vi "Dresden R2R Sputter 03.02.2018 IY24.vi"() -> ()   [LabVIEW 2009] (continued)
                                }
                                }
                                n29425 = Or(x=w34352, y=w34351) -> (x .or. y?=w34350:bool)
                                }
                                }
                                frame #1 {
                                }
                                }
                                }
                                frame #1 {
                                }
                                }
                                }
                                frame #4 {
                                n29426 = local read "Semi"() -> (w34358:bool)
                                n29427 = case shown="False" w34358 {
                                frame #0 {
                                n29428 = Wait (ms)(milliseconds to wait=u32 1000) -> ()  [unwired: 1 out]
                                }
                                frame #1 {
                                }
                                }
                                }
                                }
                                }
                                frame #1 {
                                }
                                }
                                }
                                frame #1 {
                                n29429 = local read "Semi"() -> (w34360:bool)
                                n29430 = case shown="False" w34360 {
                                frame #0 {
                                n29431 = local write "SDC1 26"(TRUE ("SDC1 26")) -> ()
                                n29432 = Wait (ms)(milliseconds to wait=u32 1000) -> ()  [unwired: 1 out]
                                }
                                frame #1 {
                                }
                                }
                                }
                                }
                                }
                                frame #23 {
                                # "sov-ar close"
                                n29433 = stacked-sequence {
                                frame #0 {
                                n29434 = local read "Semi"() -> (w34363:bool)
                                n29435 = case shown="False" w34363 {
                                frame #0 {
                                n29436 = while {
                                i -> [w34369]
                                stop <- w34364 stop-if-true
                                n29437 = Greater?(x=w34369, y=50) -> (0:w34368:bool)
                                n29438 = case shown="True" w34368 {
                                frame #0 {
                                }
                                frame #1 {
                                n29439 = local write "Semi"(TRUE ("Semi")) -> ()
                                n29440 = local write "Error Message"("Coating Process  \nwas cancelled.\nPlease check \nSOV-Ar connection." ("Error Message")) -> ()
                                }
                                }
                                n29441 = local read "Ch4_Sov_Ar_di"() -> (w34367:bool)
                                n29442 = case shown="True" w34367 {
                                tunnel: [TRUE FALSE] -> w34366
                                frame #0 {
                                }
                                frame #1 {
                                n29443 = local write "Ch4_Sov_Ar_do"(FALSE ("Ch1_WFC_do")) -> ()
                                n29444 = Wait Until Next ms Multiple(millisecond multiple=u32 200) -> ()  [unwired: 1 out]
                                }
                                }
                                n29445 = local read "Semi"() -> (w34365:bool)
                                n29446 = Or(x=w34366, y=w34365) -> (x .or. y?=w34364:bool)
                                }
                                }
                                frame #1 {
                                }
                                }
                                }
                                frame #1 {
                                n29447 = local read "Semi"() -> (w34377:bool)
                                n29448 = case shown="False" w34377 {
                                frame #0 {
                                n29449 = local write "SDC1 27"(TRUE ("SDC1 27")) -> ()
                                n29450 = Wait (ms)(milliseconds to wait=u32 1000) -> ()  [unwired: 1 out]
                                }
                                frame #1 {
                                }
                                }
                                }
                                }
                                }
                                frame #24 {
                                # "CC OPEN"
                                n29451 = stacked-sequence {
                                frame #0 {
                                n29452 = local read "Semi"() -> (w34380:bool)
                                n29453 = case shown="False" w34380 {
                                frame #0 {
                                n29454 = while {
                                i -> [w34386]
                                stop <- w34381 stop-if-true
                                n29455 = Greater?(x=w34386, y=50) -> (0:w34385:bool)
                                n29456 = case shown="True" w34385 {
                                frame #0 {
                                }
                                frame #1 {
                                n29457 = local write "Semi"(TRUE ("Semi")) -> ()
                                n29458 = local write "Error Message"("Coating Process  \nwas cancelled.\nPlease check \nBG-BV connection." ("Error Message")) -> ()
                                }
                                }
                                n29459 = local read "Ch4_Cc_on_off_di"() -> (w34384:bool)
                                n29460 = case shown="False" w34384 {
                                tunnel: [FALSE TRUE] -> w34383
                                frame #0 {
                                n29461 = local write "Ch4_Cc_on_off_do"(TRUE ("Ch1_WFC_do")) -> ()
                                n29462 = Wait Until Next ms Multiple(millisecond multiple=u32 200) -> ()  [unwired: 1 out]
                                }
                                frame #1 {
                                }
                                }
                                n29463 = local read "Semi"() -> (w34382:bool)
                                n29464 = Or(x=w34383, y=w34382) -> (x .or. y?=w34381:bool)
                                }
                                }
                                frame #1 {
                                }
                                }
                                }
                                frame #1 {
                                n29465 = local read "Semi"() -> (w34394:bool)
                                n29466 = case shown="False" w34394 {
                                frame #0 {
                                n29467 = while {
                                i -> [w34399]
                                stop <- w34397 stop-if-true
                                n29468 = Greater?(x=w34399, y=30) -> (0:w34395:bool)
                                n29469 = Wait Until Next ms Multiple(millisecond multiple=u32 1000) -> ()  [unwired: 1 out]
                                n29470 = local read "Semi"() -> (w34398:bool)
                                n29471 = Or(x=w34395, y=w34398) -> (x .or. y?=w34397:bool)
                                }
                                }
                                frame #1 {
                                }
                                }
                                }
                                frame #2 {
                                n29472 = local read "Semi"() -> (w34401:bool)
                                n29473 = case shown="False" w34401 {
                                frame #0 {
                                n29474 = local write "SDC1 27b"(TRUE ("SDC1 3")) -> ()
                                n29475 = Wait (ms)(milliseconds to wait=u32 1000) -> ()  [unwired: 1 out]
                                }
                                frame #1 {
                                }
                                }
                                }
                                }
                                }
                                frame #25 {
                                # "CHECK CHAMBER PRESSURE"
                                n29476 = stacked-sequence {
                                frame #0 {
                                n29477 = local read "Semi"() -> (w34404:bool)
                                n29478 = case shown="False" w34404 {
                                frame #0 {
                                n29479 = while {
                                i -> [w34412]
                                stop <- w34406 stop-if-true
                                n29480 = Greater?(x=w34412, y=300) -> (0:w34411:bool)
                                n29481 = case shown="True" w34411 {
                                frame #0 {
                                }
                                frame #1 {
                                n29482 = local write "Semi"(TRUE ("Semi")) -> ()
                                n29483 = local write "Error Message"("Coating Process cancelled.\nPlease check chamber \nconnections." ("Error Message")) -> ()
                                }
                                }
                                n29484 = local read "Ch_CC_press_ch4_2"() -> (w34405:dbl)
                                n29485 = Greater Or Equal?(x=w34405, y=5e-05 ("CHAMBER PRESSURE 6")) -> (x >= y?=w34409:bool)
                                n29486 = case shown="True" w34409 {
                                tunnel: [TRUE FALSE] -> w34408
                                frame #0 {
                                }
                                frame #1 {
                                n29487 = Wait Until Next ms Multiple(millisecond multiple=u32 200) -> ()  [unwired: 1 out]
                                }
                                }
                                n29488 = local read "Semi"() -> (w34407:bool)
                                n29489 = Or(x=w34408, y=w34407) -> (x .or. y?=w34406:bool)
                                }
                                }
                                frame #1 {
                                }
                                }
                                }
                                frame #1 {
                                n29490 = local read "Semi"() -> (w34419:bool)
                                n29491 = case shown="False" w34419 {
                                frame #0 {
                                n29492 = Wait (ms)(milliseconds to wait=u32 1000) -> ()  [unwired: 1 out]
                                n29493 = local write "SDC1 27c"(TRUE ("SDC1 10")) -> ()
                                }
                                frame #1 {
                                }
                                }
                                }
                                }
                                }
                                frame #26 {
                                # "encoder info  add to other web selection"
                                n29494 = stacked-sequence {
                                frame #0 {
                                n29495 = local read "Semi"() -> (w34422:bool)
                                n29496 = case shown="False" w34422 {
                                frame #0 {
                                n29497 = local read "R_Web_selection"() -> (w34423:enum32{"Web", "Other"})
                                n29498 = case shown="\"Web\", Default" w34423 {
                                frame #0 {
                                # "TC -ROLL"
                                n29499 = local read "Semi"() -> (w34424:bool)
                                n29500 = case shown="False" w34424 {
                                frame #0 {
                                n29501 = stacked-sequence {
                                frame #0 {
                                n29502 = local read "R Maximum diameter"() -> (w34426:dbl)
                                n29503 = local write "Change_Max Diameter"(w34426) -> ()
                                n29504 = Wait (ms)(milliseconds to wait=u32 300) -> ()  [unwired: 1 out]
                                }
                                frame #1 {
                                n29505 = local read "R Single RF Step1 Coating Power Active"() -> (w34427:bool)
                                n29506 = local read "R Single RF Step2 Coating Power Active"() -> (w34428:bool)
                                n29507 = local read "R Single RF Step3 Coating Power Active"() -> (w34429:bool)
                                n29508 = local read "R Single RF Step4 Coating Power Active"() -> (w34430:bool)
                                n29509 = local read "R Single RF Step5 Coating Power Active"() -> (w34431:bool)
                                n29510 = Boolean To (0,1)(Boolean=w34427) -> (0, 1=w34432:i16)
                                n29511 = Boolean To (0,1)(Boolean=w34428) -> (0, 1=w34433:i16)
                                n29512 = Boolean To (0,1)(Boolean=w34429) -> (0, 1=w34434:i16)
                                n29513 = Boolean To (0,1)(Boolean=w34430) -> (0, 1=w34435:i16)
                                n29514 = Boolean To (0,1)(Boolean=w34431) -> (0, 1=w34436:i16)
                                n29515 = Compound Arithmetic op=ADD(w34432, w34433, w34434, w34435, w34436) -> (w34438:i16)
                                n29516 = local read "R Single RF Interval length"() -> (w34437:dbl)
                                n29517 = Multiply(x=w34437, y=w34438) -> (x*y=w34439:dbl)
                                n29518 = local write "Total length"(w34439) -> ()
                                }
                                frame #2 {
                                n29519 = local write "Calculate 3"(TRUE ("Calculate_auto")) -> ()
                                }
                                frame #3 {
                                n29520 = Wait (ms)(milliseconds to wait=u32 1000) -> ()  [unwired: 1 out]
                                }
                                frame #4 {
                                n29521 = local read "Change_Max Diameter"() -> (w34444:dbl)
                                n29522 = Wait (ms)(milliseconds to wait=u32 200) -> ()  [unwired: 1 out]
                                n29523 = local write "Web Speed"(200.0 ("Web Speed")) -> ()
                                n29524 = local write "Initial Min Diameter"(w34444) -> ()
                                }
                                frame #5 {
                                n29525 = local write "Calculate 2"(TRUE ("Calculate_auto")) -> ()
                                }
                                frame #6 {
                                n29526 = local write "Roll_side_select"(enum32{"Left to Right", "Right to Left"}."Right to Left" ("Roll_side_select")) -> ()
                                }
                                frame #7 {
                                n29527 = Wait (ms)(milliseconds to wait=u32 100) -> ()  [unwired: 1 out]
                                n29528 = local write "Parameters_auto_set"(TRUE ("Parameters_auto_set")) -> ()
                                }
                                frame #8 {
                                n29529 = while {
                                i -> [w34453]
                                stop <- w34449 stop-if-true
                                n29530 = Wait Until Next ms Multiple(millisecond multiple=u32 300) -> ()  [unwired: 1 out]
                                n29531 = Greater?(x=w34453, y=100) -> (0:w34450:bool)
                                n29532 = local read "Parameters_auto_set"() -> (w34454:bool)
                                n29533 = case shown="False" w34454 {
                                tunnel: [TRUE FALSE] -> w34451
                                frame #0 {
                                }
                                frame #1 {
                                }
                                }
                                n29534 = Or(x=w34451, y=w34450) -> (x .or. y?=w34449:bool)
                                }
                                }
                                frame #9 {
                                n29535 = local read "R Tension Value"() -> (w34458:dbl)
                                n29536 = Wait (ms)(milliseconds to wait=u32 200) -> ()  [unwired: 1 out]
                                n29537 = local write "TC2_set_value"(w34458) -> ()
                                }
                                frame #10 {
                                n29538 = local write "TC2_auto_set"(TRUE ("TC1_auto_set")) -> ()
                                }
                                frame #11 {
                                w34461 = u16 3 items=["1", "2", "3", "4"] ("Target Chamber Sensor")
                                n29539 = local write "Target Chamber Sensor"(w34461) -> ()
                                }
                                frame #12 {
                                n29540 = local read "Total length"() -> (w34462:dbl)
                                n29541 = local write "Region"(w34462) -> ()
                                }
                                frame #13 {
                                n29542 = local read "Semi"() -> (w34463:bool)
                                n29543 = case shown="False" w34463 {
                                frame #0 {
                                n29544 = local write "Start_roll"(TRUE ("Start_roll")) -> ()
                                n29545 = Wait (ms)(milliseconds to wait=u32 300) -> ()  [unwired: 1 out]
                                }
                                frame #1 {
                                }
                                }
                                }
                                frame #14 {
                                n29546 = local read "Semi"() -> (w34466:bool)
                                n29547 = case shown="False" w34466 {
                                frame #0 {
                                n29548 = while {
                                stop <- w34470 stop-if-true
                                n29549 = Wait Until Next ms Multiple(millisecond multiple=u32 200 ("milliseconds to wait")) -> ()  [unwired: 1 out]
                                n29550 = local read "Start_roll"() -> (w34468:bool)
                                n29551 = Not(x=w34468) -> (.not. x?=w34467:bool)
                                n29552 = local read "Semi"() -> (w34471:bool)
                                n29553 = Or(x=w34467, y=w34471) -> (x .or. y?=w34470:bool)
                                }
                                }
                                frame #1 {
                                }
                                }
                                }
                                }
                                }
                                frame #1 {
                                }
                                }
                                }
                                frame #1 {
                                n29554 = disable-structure shown="Disabled" {
                                frame #0 {
                                # "OTHER"
                                n29555 = local read "Semi"() -> (w34472:bool)
                                n29556 = case shown="False" w34472 {
                                frame #0 {
                                n29557 = stacked-sequence {
                                frame #0 {
                                n29558 = local read "Semi"() -> (w34473:bool)
                                n29559 = case shown="False" w34473 {
                                frame #0 {
                                n29560 = while {
                                i -> [w34479]
                                stop <- w34476 stop-if-true
                                n29561 = Greater?(x=w34479, y=50) -> (0:w34478:bool)
                                n29562 = case shown="True" w34478 {
                                frame #0 {
                                }
                                frame #1 {
                                n29563 = local write "Error Message"("" ("Error Message")) -> ()
                                n29564 = local write "Semi"(TRUE ("Semi")) -> ()
                                }
                                }
                                n29565 = local read "Casette_servo_start/stop_di"() -> (w34475:bool)
                                n29566 = case shown="False" w34475 {
                                tunnel: [FALSE TRUE] -> w34474
                                frame #0 {
                                n29567 = local write "Casette_servo_start/stop_do"(TRUE ("Casette_servo_left_direction_do")) -> ()
                                n29568 = Wait Until Next ms Multiple(millisecond multiple=u32 500) -> ()  [unwired: 1 out]
                                }
                                frame #1 {
                                }
                                }
                                n29569 = local read "Semi"() -> (w34477:bool)
                                n29570 = Or(x=w34474, y=w34477) -> (x .or. y?=w34476:bool)
                                }
                                }
                                frame #1 {
                                }
                                }
                                }
                                frame #1 {
                                n29571 = local read "Semi"() -> (w34487:bool)
                                n29572 = case shown="False" w34487 {
                                frame #0 {
                                n29573 = while {
                                i -> [w34493]
                                stop <- w34490 stop-if-true
                                n29574 = Greater?(x=w34493, y=50) -> (0:w34492:bool)
                                n29575 = case shown="True" w34492 {
                                frame #0 {
                                }
                                frame #1 {
                                n29576 = local write "Error Message"("" ("Error Message")) -> ()
                                n29577 = local write "Semi"(TRUE ("Semi")) -> ()
                                }
                                }
                                n29578 = local read "Casette_servo_left_direction_di"() -> (w34489:bool)
                                n29579 = case shown="False" w34489 {
                                tunnel: [FALSE TRUE] -> w34488
                                frame #0 {
                                n29580 = local write "Casette_servo_left_direction_do"(TRUE ("Casette_servo_left_direction_do")) -> ()
                                n29581 = Wait Until Next ms Multiple(millisecond multiple=u32 200) -> ()  [unwired: 1 out]
                                }
                                frame #1 {
                                }
                                }
                                n29582 = local read "Semi"() -> (w34491:bool)
                                n29583 = Or(x=w34488, y=w34491) -> (x .or. y?=w34490:bool)
                                }
                                }
                                frame #1 {
                                }
                                }
                                }
                                frame #2 {
                                # "casette motion"
                                n29584 = while {
                                i -> [w34503]
                                stop <- w34501 stop-if-true
                                n29585 = Greater?(x=w34503, y=200) -> (0:w34504:bool)
                                n29586 = case shown="True" w34504 {
                                frame #0 {
                                }
                                frame #1 {
                                n29587 = local write "Semi"(TRUE ("Semi")) -> ()
                                }
                                }
                                n29588 = local read "Counter_read_data"() -> (w34509:i16)
                                n29589 = Greater?(x=w34509, y=i16 0) -> (0:w34507:bool)
                                n29590 = case shown="True" w34507 {
                                tunnel: [TRUE TRUE] -> w34506
                                frame #0 {
                                }
                                frame #1 {
                                n29591 = local write "Casette_servo_start/stop_do"(FALSE ("Casette_servo_start/stop_do")) -> ()
                                n29592 = Wait Until Next ms Multiple(millisecond multiple=u32 200) -> ()  [unwired: 1 out]
                                }
                                }
                                n29593 = local read "Semi"() -> (w34505:bool)
                                n29594 = Or(x=w34506, y=w34505) -> (x .or. y?=w34501:bool)
                                }
                                }
                                frame #3 {
                                n29595 = local read "Semi"() -> (w34515:bool)
                                n29596 = case shown="False" w34515 {
                                frame #0 {
                                n29597 = while {
                                i -> [w34521]
                                stop <- w34518 stop-if-true
                                n29598 = Greater?(x=w34521, y=50) -> (0:w34520:bool)
                                n29599 = case shown="True" w34520 {
                                frame #0 {
                                }
                                frame #1 {
                                n29600 = local write "Error Message"("" ("Error Message")) -> ()
                                n29601 = local write "Semi"(TRUE ("Semi")) -> ()
                                }
                                }
                                n29602 = local read "Casette_servo_start/stop_di"() -> (w34517:bool)
                                n29603 = case shown="True" w34517 {
                                tunnel: [TRUE FALSE] -> w34516
                                frame #0 {
                                }
                                frame #1 {
                                n29604 = local write "Casette_servo_start/stop_do"(FALSE ("Casette_servo_left_direction_do")) -> ()
                                n29605 = Wait Until Next ms Multiple(millisecond multiple=u32 500) -> ()  [unwired: 1 out]
                                }
                                }
                                n29606 = local read "Semi"() -> (w34519:bool)
                                n29607 = Or(x=w34516, y=w34519) -> (x .or. y?=w34518:bool)
                                }
                                }
                                frame #1 {
                                }
                                }
                                }
                                frame #4 {
                                n29608 = local read "Semi"() -> (w34529:bool)
                                n29609 = case shown="False" w34529 {
                                frame #0 {
                                n29610 = Wait Until Next ms Multiple(millisecond multiple=u32 5000 ("millisecond multiple 9")) -> ()  [unwired: 1 out]
                                }
                                frame #1 {
                                }
                                }
                                }
                                frame #5 {
                                n29611 = local read "Semi"() -> (w34531:bool)
                                n29612 = case shown="False" w34531 {
                                frame #0 {
                                n29613 = while {
                                i -> [w34537]
                                stop <- w34534 stop-if-true
                                n29614 = Greater?(x=w34537, y=50) -> (0:w34536:bool)
                                n29615 = case shown="True" w34536 {
                                frame #0 {
                                }
                                frame #1 {
                                n29616 = local write "Error Message"("" ("Error Message")) -> ()
                                n29617 = local write "Semi"(TRUE ("Semi")) -> ()
                                }
                                }
                                n29618 = local read "Casette_servo_start/stop_di"() -> (w34533:bool)
                                n29619 = case shown="False" w34533 {
                                tunnel: [FALSE TRUE] -> w34532
                                frame #0 {
                                n29620 = local write "Casette_servo_start/stop_do"(TRUE ("Casette_servo_left_direction_do")) -> ()
                                n29621 = Wait Until Next ms Multiple(millisecond multiple=u32 500) -> ()  [unwired: 1 out]
                                }
                                frame #1 {
                                }
                                }
                                n29622 = local read "Semi"() -> (w34535:bool)
                                n29623 = Or(x=w34532, y=w34535) -> (x .or. y?=w34534:bool)
                                }
                                }
                                frame #1 {
                                }
                                }
                                }
                                frame #6 {
                                n29624 = local read "Semi"() -> (w34545:bool)
                                n29625 = case shown="False" w34545 {
                                frame #0 {
                                n29626 = while {
                                i -> [w34551]
                                stop <- w34548 stop-if-true
                                n29627 = Greater?(x=w34551, y=50) -> (0:w34550:bool)
                                n29628 = case shown="True" w34550 {
                                frame #0 {
                                }
                                frame #1 {
                                n29629 = local write "Error Message"("" ("Error Message")) -> ()
                                n29630 = local write "Semi"(TRUE ("Semi")) -> ()
                                }
                                }
                                n29631 = local read "Casette_servo_left_direction_di"() -> (w34547:bool)
                                n29632 = case shown="True" w34547 {
                                tunnel: [TRUE FALSE] -> w34546
                                frame #0 {
                                }
                                frame #1 {
                                n29633 = local write "Casette_servo_left_direction_do"(FALSE ("Casette_servo_left_direction_do")) -> ()
                                n29634 = Wait Until Next ms Multiple(millisecond multiple=u32 200) -> ()  [unwired: 1 out]
                                }
                                }
                                n29635 = local read "Semi"() -> (w34549:bool)
                                n29636 = Or(x=w34546, y=w34549) -> (x .or. y?=w34548:bool)
                                }
                                }
                                frame #1 {
                                }
                                }
                                }
                                frame #7 {
                                # "casette motion"
                                n29637 = while {
                                i -> [w34562]
                                stop <- w34559 stop-if-true
                                n29638 = Greater?(x=w34562, y=200) -> (0:w34563:bool)
                                n29639 = case shown="True" w34563 {
                                frame #0 {
                                }
                                frame #1 {
                                n29640 = local write "Semi"(TRUE ("Semi")) -> ()
                                }
                                }
                                n29641 = local read "Counter_read_data"() -> (w34567:i16)
                                n29642 = Less?(x=w34567, y=i16 0) -> (x < y?=w34566:bool)
                                n29643 = case shown="True" w34566 {
                                tunnel: [TRUE TRUE] -> w34565
                                frame #0 {
                                }
                                frame #1 {
                                n29644 = local write "Casette_servo_start/stop_do"(FALSE ("Casette_servo_start/stop_do")) -> ()
                                n29645 = Wait Until Next ms Multiple(millisecond multiple=u32 200) -> ()  [unwired: 1 out]
                                }
                                }
                                n29646 = local read "Semi"() -> (w34564:bool)
                                n29647 = Or(x=w34565, y=w34564) -> (x .or. y?=w34559:bool)
                                }
                                }
                                frame #8 {
                                n29648 = local read "Semi"() -> (w34573:bool)
                                n29649 = case shown="False" w34573 {
                                frame #0 {
                                n29650 = while {
                                i -> [w34579]
                                stop <- w34576 stop-if-true
                                n29651 = Greater?(x=w34579, y=50) -> (0:w34578:bool)
                                n29652 = case shown="True" w34578 {
                                frame #0 {
                                }
                                frame #1 {
                                n29653 = local write "Error Message"("" ("Error Message")) -> ()
                                n29654 = local write "Semi"(TRUE ("Semi")) -> ()
                                }
                                }
                                n29655 = local read "Casette_servo_start/stop_di"() -> (w34575:bool)
                                n29656 = case shown="True" w34575 {
                                tunnel: [TRUE FALSE] -> w34574
                                frame #0 {
                                }
                                frame #1 {
                                n29657 = local write "Casette_servo_start/stop_do"(FALSE ("Casette_servo_left_direction_do")) -> ()
                                n29658 = Wait Until Next ms Multiple(millisecond multiple=u32 500) -> ()  [unwired: 1 out]
                                }
                                }
                                n29659 = local read "Semi"() -> (w34577:bool)
                                n29660 = Or(x=w34574, y=w34577) -> (x .or. y?=w34576:bool)
                                }
                                }
                                frame #1 {
                                }
                                }
                                }
                                frame #9 {
                                n29661 = local read "Semi"() -> (w34587:bool)
                                n29662 = case shown="False" w34587 {
                                frame #0 {
                                }
                                frame #1 {
                                }
                                }
                                }
                                }
                                }
                                frame #1 {
                                }
                                }
                                }
                                frame #1 {
                                }
                                }
                                }
                                }
                                }
                                frame #1 {
                                }
                                }
                                }
                                frame #1 {
                                n29663 = local read "Semi"() -> (w34588:bool)
                                n29664 = case shown="False" w34588 {
                                frame #0 {
                                n29665 = Wait (ms)(milliseconds to wait=u32 1000) -> ()  [unwired: 1 out]
                                n29666 = local write "SDC1 29"(TRUE ("SDC1 29")) -> ()
                                }
                                frame #1 {
                                }
                                }
                                }
                                }
                                }
                                frame #27 {
                                n29667 = local read "Semi"() -> (w34591:bool)
                                n29668 = case shown="False" w34591 {
                                frame #0 {
                                n29669 = local write "Cnt_Do_Buzzer"(TRUE ("SDC1 30")) -> ()
                                n29670 = Wait (ms)(milliseconds to wait=u32 2500) -> ()  [unwired: 1 out]
                                n29671 = local write "SDC1 30"(TRUE ("SDC1 30")) -> ()
                                }
                                frame #1 {
                                }
                                }
                                }
                                frame #28 {
                                n29672 = local read "Semi"() -> (w34595:bool)
                                n29673 = case shown="False" w34595 {
                                frame #0 {
                                n29674 = local write "Cnt_Do_Buzzer"(FALSE ("SDC1 30")) -> ()
                                n29675 = Wait (ms)(milliseconds to wait=u32 1000) -> ()  [unwired: 1 out]
                                }
                                frame #1 {
                                }
                                }
                                }
                                }
                                }
                                frame #1 {
                                }
                              }
                            }
                          }
                        }
                      }
                    }
                    frame #1 {
                      n29676 = local read "Ch2_pressure"() -> (w34608:dbl)
                      n29677 = local read "Ch3_pressure"() -> (w34603:dbl)
                      n29678 = local read "started_up_ch2"() -> (w34601:bool)
                      n29679 = local read "started_up_ch3"() -> (w34599:bool)
                      n29680 = In Range and Coerce(upper limit="MW_Coating_Interlock 5", x=w34608, lower limit=1e-08) -> (In Range?=w34602:bool)  [unwired: 1 out]
                      n29681 = In Range and Coerce(upper limit="MW_Coating_Interlock 6", x=w34603, lower limit=1e-08) -> (In Range?=w34600:bool)  [unwired: 1 out]
                      n29682 = Compound Arithmetic op=AND(w34602, w34601, w34600, w34599) -> (w34598:bool)
                      n29683 = case shown="True" w34598 {
                        frame #0 {
                        }
                        frame #1 {
                          n29684 = stacked-sequence {
                            frame #0 {
                              n29685 = while {
                                i -> [w34614]
                                stop <- w34612 stop-if-true
                                n29686 = local read "R Cmb Number of pairs"() -> (w34611:dbl)
                                n29687 = Greater Or Equal?(x=w34614, y=w34611) -> (x >= y?=w34610:bool)
                                n29688 = case shown="False" w34610 {
                                tunnel: [FALSE TRUE] -> w34609
                                frame #0 {
                                n29689 = stacked-sequence {
                                frame #0 {
                                n29690 = local read "Single_ch3_Interlock"() -> (w34616:dbl)
                                n29691 = local read "Ch3_pressure"() -> (w34620:dbl)
                                n29692 = local read "started_up_ch3"() -> (w34618:bool)
                                n29693 = In Range and Coerce(upper limit=w34616, x=w34620, lower limit=1e-08) -> (In Range?=w34621:bool)  [unwired: 1 out]
                                n29694 = And(x=w34621, y=w34618) -> (x .and. y?=w34617:bool)
                                n29695 = case shown="True" w34617 {
                                frame #0 {
                                }
                                frame #1 {
                                n29696 = local read "Semi"() -> (w34622:bool)
                                n29697 = case shown="False" w34622 {
                                frame #0 {
                                n29698 = stacked-sequence {
                                frame #0 {
                                n29699 = local read "ch_present_position"() -> (w34625:dbl)
                                n29700 = Not Equal?(x=w34625, y=3.0) -> (x != y?=w34623:bool)
                                n29701 = case shown="True" w34623 {
                                frame #0 {
                                }
                                frame #1 {
                                n29702 = stacked-sequence {
                                frame #0 {
                                n29703 = local write "Set chamber"(3.0 ("Set chamber")) -> ()
                                n29704 = Wait (ms)(milliseconds to wait=u32 100) -> ()  [unwired: 1 out]
                                }
                                frame #1 {
                                n29705 = local write "Auto_set_transfer"(TRUE ("Auto_set_transfer")) -> ()
                                }
                                frame #2 {
                                n29706 = while {
                                stop <- w34630 stop-if-true
                                n29707 = Wait Until Next ms Multiple(millisecond multiple=u32 300) -> ()  [unwired: 1 out]
                                n29708 = local read "Auto_set_transfer"() -> (w34631:bool)
                                n29709 = local read "Semi"() -> (w34633:bool)
                                n29710 = Not(x=w34631) -> (.not. x?=w34632:bool)
                                n29711 = Or(x=w34632, y=w34633) -> (x .or. y?=w34630:bool)
                                }
                                }
                                frame #3 {
                                n29712 = Wait (ms)(milliseconds to wait=u32 300) -> ()  [unwired: 1 out]
                                n29713 = local write "SCMB0 2"(TRUE ("SMW1 2")) -> ()
                                }
                                }
                                }
                                }
                                }
                                frame #1 {
                                # "WATER FLOW CONTROL OPEN"
                                n29714 = stacked-sequence {
                                frame #0 {
                                n29715 = local read "Semi"() -> (w34636:bool)
                                n29716 = case shown="False" w34636 {
                                frame #0 {
                                n29717 = while {
                                i -> [w34642]
                                stop <- w34637 stop-if-true
                                n29718 = Greater?(x=w34642, y=100) -> (0:w34641:bool)
                                n29719 = case shown="True" w34641 {
                                frame #0 {
                                }
                                frame #1 {
                                n29720 = local write "Semi"(TRUE ("Semi")) -> ()
                                n29721 = local write "Error Message"("Coating Process  \nwas cancelled.\nPlease check water \nflow connection." ("Error Message")) -> ()
                                }
                                }
                                n29722 = local read "Ch4_WFS_di"() -> (w34640:bool)
                                n29723 = case shown="True" w34640 {
                                tunnel: [TRUE FALSE] -> w34639
                                frame #0 {